vi "HFRR ADV v039 new software.vi"() -> ()   [LabVIEW 2025] (continued)
    n1685 = Fract/Exp String To Number(string=w2065) -> (number=w2064:dbl[])  [unwired: 3 in, 1 out]
    n1686 = call <vilib>:"Median Filter PtByPt.vi"("rank"=2, "x"=w2050) -> ("Filtered x"=→"Friction":dbl)  [unwired: 2 in, 1 out]
    n1687 = Index Array(array=w2064) -> (element #1=→"Sample Temperature":dbl, element #2=→"Target Sample Temperature":dbl, element #3=→"Current Duty Cycle":dbl, element #4=→"Ambient Temperature":dbl, element #5=→"Dac Status":dbl, element #6=→"Vpp":dbl, element #7=→"Active Error Code":dbl, element #8=→"Kp":dbl, element #9=→"Ki":dbl, element #10=→"Kd":dbl, element #11=→"SampleRaw":dbl, element #12=→"AmbRaw":dbl)  [unwired: 12 in]
    n1688 = local read "Quit"() -> (w2070:bool)
  }
  n1689 = while {
    shift-right: [w2084] -> w41
    shift-left: _ -> [w2076]
    shift-right: [w2071] -> w40
    shift-left: errorcluster {"status"=FALSE, "code"=0, "source"="Init"} ("error out") -> [w2078]
    tunnel: [w2073] -> w44
    tunnel: [w2083] -> _
    i -> [w2083]
    stop <- w2073 stop-if-true
    n1690 = local read "Com Port 2"() -> (w2077:refnum<visa-resource-name>)
    n1691 = local read "Port 2a"() -> (w2079:bool)
    n1692 = Unbundle(w2078) -> ("status"=→"Port 4":bool)  [unwired: 2 out]
    n1693 = call <vilib>:"High Resolution Polling Wait.vi"("seconds to wait"=0.02) -> ()  [unwired: 10 in, 1 out]
    n1694 = local read "Port 4"() -> (w2080:bool)
    n1695 = Not Equal?(x=w2077, y=w2076) -> (x != y?=w2075:bool)
    n1696 = Or(x=w2080, y=w2079) -> (x .or. y?=w2082:bool)
    n1697 = case shown="False" w2082 {
      frame False {
        w2087 = TRUE ("Visible")
        n1698 = property on="Port 2a" class="Bool (strict)"("Visible"=w2087) -> ()  [unwired: 2 in, 2 out]
        n1699 = property on="Port 4" class="Bool (strict)"("Visible"=w2087) -> ()  [unwired: 2 in, 2 out]
      }
      frame True {
        w2088 = TRUE ("Visible")
        n1700 = property on="Port 2a" class="Bool (strict)"("Visible"=w2088) -> ()  [unwired: 2 in, 2 out]
        n1701 = property on="Port 4" class="Bool (strict)"("Visible"=w2088) -> ()  [unwired: 2 in, 2 out]
      }
    }
    n1702 = case shown="True" w2075 {
      tunnel: [w2085 errorcluster {"status"=TRUE, "code"=0, "source"="Init"} ("error out")] -> w2074
      tunnel: w2078 -> [w2085 _]
      frame False {
      }
      frame True {
      }
    }
    n1703 = case shown="No Error" w2074 {
      selector: w2074 -> [w2101 w2132]
      tunnel: [w2094 w2137] -> w2084
      tunnel: [w2102 w2130] -> w2071
      tunnel: w2076 -> [w2103 w2135]
      frame No Error {
        n1704 = property class="Instr" props=["Serial Settings:Number of Bytes at Serial Port"](reference=w2103, error in=w2101) -> (reference out=w2095:refnum<visa-resource-name>, error out=w2100:errorcluster)  [unwired: 1 out]
        n1705 = while {
          tunnel: [w2111] -> w2096
          tunnel: [w2110] -> w2097
          tunnel: w2100 -> [w2109]
          tunnel: w2095 -> [w2108]
          tunnel: [w2107] -> _
          i -> [w2107]
          stop <- TRUE stop-if-true
          n1706 = property class="Instr" props=["Serial Settings:Number of Bytes at Serial Port"](reference=w2108, error in=w2109) -> (reference out=w2113:refnum<visa-resource-name>, error out=w2112:errorcluster)  [unwired: 1 out]
          n1707 = VISA Read(VISA resource name=w2113, byte count=u32 1000, error in (no error)=w2112) -> (VISA resource name out=w2110:refnum<visa-resource-name>, read buffer=→"Due read":string, error out=w2111:errorcluster)  [unwired: 1 out]
        }
        n1708 = local read "Due Write"() -> (w2093:string)
        n1709 = call <vilib>:"Trim Whitespace.vi"("string"=w2093) -> ("trimmed string"=w2092:string)  [unwired: 1 in]
        n1710 = Not Equal?(x=w2092, y="") -> (x != y?=w2098:bool)
        n1711 = VISA Flush I/O Buffer(VISA resource name=w2097) -> (VISA resource name out=w2090:refnum<visa-resource-name>, error out=→"error out 10":errorcluster)  [unwired: 2 in]
        n1712 = case shown="True" w2098 {
          tunnel: w2090 -> [w2115 w2120]
          tunnel: [w2115 w2124] -> w2094
          tunnel: w2096 -> [w2114 w2119]
          tunnel: [w2114 w2122] -> w2102
          tunnel: w2092 -> [_ w2118]
          tunnel: [_ w2121] -> _
          frame False {
            # "DATA  WRITE LOOP"
          }
          frame True {
            n1713 = Concatenate Strings(w2118, "\r\n") -> (w2117:string)
            n1714 = VISA Write(VISA resource name=w2120, write buffer=w2117, error in (no error)=w2119) -> (VISA resource name out=w2124:refnum<visa-resource-name>, return count=w2121:u32, error out=w2123:errorcluster)
            n1715 = flat-sequence {
              tunnel: w2123 -> [w2126]
              tunnel: [w2126] -> w2122
              frame #0 {
                n1716 = local write "Due Write"("" ("Command")) -> ()
                n1717 = Wait (ms)(milliseconds to wait=u32 5) -> ()  [unwired: 1 out]
              }
            }
          }
        }
        "Port 2a" <- TRUE ("Port 2a")
      }
      frame Error {
        w2143 = u16 0 items=["None", "XON/XOFF", "RTS/CTS", "XON/XOFF & RTS/CTS", "DTR/DSR", "XON/XOFF & DTR/DSR"] ("flow control (0:none)  2")
        w2141 = u16 10 items=["1.0"=10, "1.5"=15, "2.0"=20] ("stop bits 2")
        w2139 = u16 0 items=["None", "Odd", "Even", "Mark", "Space"] ("parity 2")
        w2140 = u32 10000  # timeout (10sec)
        n1718 = VISA Clear(VISA resource name=w2135, error in (no error)=w2132) -> (VISA resource name out=w2134:refnum<visa-resource-name>, error out=w2133:errorcluster)
        n1719 = VISA Close(VISA resource name=w2134, error in (no error)=w2133) -> (error out=w2136:errorcluster)
        n1720 = call <vilib>:"Clear Errors.vi"("error in (no error)"=w2136) -> ()  [unwired: 5 in, 2 out]
        n1721 = local write "Port 2a"(FALSE ("Port 2a")) -> ()
        n1722 = local read "Com Port 2"() -> (w2129:refnum<visa-resource-name>)
        "visa due" <- w2129
        n1723 = call-poly "VISA Configure Serial Port"("VISA resource name"=w2129, "timeout (10sec)"=w2140, "baud rate (9600)"=u32 250000 ("baud rate  2"), "data bits (8)"=u16 8 ("data bits  2"), "parity (0:none)"=w2139, "stop bits (10: 1 bit)"=w2141, "flow control (0:none)"=w2143) -> ("VISA resource name out"=w2144:refnum<visa-resource-name>, "error out"=w2145:errorcluster)  [unwired: 7 in]
        n1724 = flat-sequence {
          tunnel: w2144 -> [w2147]
          tunnel: w2145 -> [w2146]
          tunnel: [w2147] -> w2137
          tunnel: [w2146] -> w2130
          frame #0 {
            n1725 = Wait (ms)(milliseconds to wait=u32 50) -> ()  [unwired: 1 out]
          }
        }
        "Residual Due" <- ""
      }
    }
    "error out 9" <- w2071
    n1726 = local read "Quit"() -> (w2073:bool)
    "Error Due" <- w2078
  }
  n1727 = local write "FRICVALZ"(0.0 ("FRICVALZ")) -> ()
  n1728 = property on="RUN" class="Bool (strict)"("Visible"=TRUE) -> ()  [unwired: 2 in, 2 out]
  n1729 = while {
    tunnel: [w2162] -> _
    tunnel: [w2149] -> w54
    i -> [w2162]
    stop <- w2149 stop-if-true
    # "DATA PROCESSING"
    # "115 mV/N"
    n1730 = local read "conststatus"() -> (w2153:dbl)
    n1731 = local read "Main Tab"() -> (w2151:T2)
    n1732 = local read "EDIT"() -> (w2168:bool)
    n1733 = local read "Rate"() -> (w2167:dbl)
    n1734 = case shown="True" w2168 {
      tunnel: [FALSE TRUE] -> _
      frame False {
      }
      frame True {
      }
    }
    n1735 = Equal?(x=w2151, y=T29."About" ("Main Tab")) -> (x = y?=w2160:bool)
    n1736 = Equal?(x=w2153, y=0.0) -> (x = y?=w2154:bool)
    n1737 = Divide(x=1.0, y=w2167) -> (x/y=w2163:dbl)
    "Time 2" <- w2163
    n1738 = case shown="True" w2154 {
      frame False {
      }
      frame True {
        # "C:\\WinDucom\\calibrate WO 2391.dcf"
        n1739 = local write "Lan flag"(22) -> ()
        n1740 = local write "conststatus"(10.0 ("rpm value : 2")) -> ()
        n1741 = String To Path(string="C:\\LAB-IQ\\calibrate WO 2465.dcf") -> (path=w2174:path)
        n1742 = Open/Create/Replace File "Open File"(file path (use dialog)=w2174) -> (refnum out=w2172:refnum<file>)  [unwired: 5 in, 2 out]
        n1743 = for {
          N: 23 -> [_]
          tunnel: w2172 -> [w2183]
          i -> [w2177]
          (unwired) TRUE ("line mode (F)")
          n1744 = Read from Text File "Read File"(file (use dialog)=w2183) -> (text=w2182:string)  [unwired: 3 in, 3 out]
          n1745 = Match Pattern(string=w2182, regular expression="]") -> (after substring=w2180:string)  [unwired: 1 in, 3 out]
          n1746 = String Subset(string=w2182, offset (0)=5, length (rest)=10 ("length (rest)")) -> (substring=w2175:string)
          n1747 = Fract/Exp String To Number(string=w2175) -> (number=w2176:dbl)  [unwired: 3 in, 1 out]
          n1748 = Match Pattern(string=w2180, regular expression="-") -> (before substring=w2178:string)  [unwired: 1 in, 3 out]
          n1749 = case shown="10" w2177 {
            tunnel: w2176 -> [_ _ _ _ _ _ _ _ _ _ w2190 _ _ _ _ _ _ _ _ _ _ _ _ _]
            tunnel: w2178 -> [_ _ _ _ w2186 w2187 w2188 _ _ _ _ _ _ _ _ _ _ _ _ _ w2191 w2192 w2193 _]
            frame 0 {
            }
            frame 1 {
            }
            frame 2 {
            }
            frame 3 {
            }
            frame 4 {
              n1750 = local write "Com Port 1"(w2186) -> ()
            }
            frame 5 {
              n1751 = local write "Com Port 2"(w2187) -> ()
              n1752 = local write "visa due"(w2187) -> ()
            }
            frame 6 {
              n1753 = String To Path(string=w2188) -> (path=w2189:path)
              n1754 = local write "File Path"(w2189) -> ()
              "String" <- w2188
            }
            frame 7 {
            }
            frame 8 {
            }
            frame 9 {
            }
            frame 10 {
              n1755 = local write "Language Selection"(w2190) -> ()
            }
            frame 11 {
            }
            frame 12 {
            }
            frame 13 {
            }
            frame 14 {
            }
            frame 15 {
            }
            frame 16 {
            }
            frame 17 {
            }
            frame 18 {
            }
            frame 21 {
            }
            frame 22 {
              n1756 = local write "Com Port 3"(w2191) -> ()
            }
            frame 20 {
              n1757 = local write "Camera Port :"(w2192) -> ()
            }
            frame 19 {
              n1758 = local write "C3 :"(w2193) -> ()
            }
            frame 23, Default {
            }
          }
        }
      }
    }
    n1759 = Select(t=u32 2500 ("milliseconds to wait"), s=w2160, f=u32 500 ("milliseconds to wait")) -> (s? t:f=w2158:u32)
    n1760 = Multiply(x=w2163, y=w2158) -> (x*y=w2165:dbl)
    n1761 = call "Elapsed Time2"("Time Target (s)"=w2165, "Auto Reset"=TRUE) -> ("Time has Elapsed"=w2155:bool)  [unwired: 10 in, 7 out]
    n1762 = case shown="True" w2155 {
      frame False {
      }
      frame True {
        n1763 = stacked-sequence {
          frame #0 {
            n1764 = local read "Sample Temperature"() -> (w2197:dbl)
            n1765 = local read "RH Numeric:"() -> (→"Humidity ( %RH )" →"Hum":dbl)
            n1766 = local read "FF CONTINUE 5"() -> (w2194:bool)
            n1767 = local read "FRICVALZ"() -> (w2214:dbl)
            n1768 = local read "Friction"() -> (w2200:dbl)
            n1769 = call <vilib>:"Mean PtByPt.vi"("x"=w2197, "sample length"=100) -> ("mean"=w2196:dbl)  [unwired: 2 in, 1 out]
            "TEMP 2" <- w2196
            "TEMP 3" <- w2196
            n1770 = Subtract(x=w2200, y=w2214) -> (x-y=w2209:dbl)
            "FF 2" <- w2209
            "FF 4" <- w2209
            n1771 = local read "Ambient Temperature"() -> (→"AIR TEMP":dbl)
            n1772 = local read "TEMP"() -> (w2213:dbl)
            n1773 = local write "FF 3"(w2209) -> ()
            n1774 = Compound Arithmetic op=OR("FRICVALZ 4", "FRICVALZ 3", "FRICVALZ 2", w2194) -> (w2205:bool)
            n1775 = case shown="True" w2205 {
              tunnel: w2200 -> [_ w2220]
              frame False {
              }
              frame True {
                w2219 = FALSE ("FRICVALZ")
                n1776 = local write "FRICVALZ 3"(w2219) -> ()
                n1777 = local write "FRICVALZ 2"(w2219) -> ()
                n1778 = local write "FRICVALZ 4"(w2219) -> ()
                n1779 = local write "FF CONTINUE 5"(w2219) -> ()
                "FRICVALZ" <- w2220
              }
            }
            n1780 = Not A Number/Path/Refnum?(number/path/refnum=w2213) -> (NaN/Path/Refnum?=w2212:bool)
            n1781 = Not A Number/Path/Refnum?(number/path/refnum=w2209) -> (NaN/Path/Refnum?=w2211:bool)
            n1782 = Divide(x=w2209, y=1.96) -> (x/y=w2206:dbl)
            n1783 = Compound Arithmetic op=OR(w2212, w2211) -> (w2210:bool)
            n1784 = Not A Number/Path/Refnum?(number/path/refnum=w2206) -> (NaN/Path/Refnum?=w2207:bool)
            n1785 = case shown="True" w2210 {
              frame False {
              }
              frame True {
                n1786 = local write "TEMP"(0.0 ("TEMP")) -> ()
                n1787 = local write "FF 2"(0.0 ("FF 2")) -> ()
                n1788 = local write "reinit"(TRUE ("reinit")) -> ()
              }
            }
            n1789 = local write "TEMP"(w2196) -> ()
            n1790 = Select(t=0.0, s=w2207, f=w2206) -> (s? t:f=w2199:dbl)
            "COF 2" <- w2199
            n1791 = local write "COF 3"(w2199) -> ()
          }
        }
      }
    }
    n1792 = Wait (ms)(milliseconds to wait=u32 50) -> ()  [unwired: 1 out]
    n1793 = local read "Quit"() -> (w2149:bool)
    "Rate" <- 2500.0 ("No of Samples")
  }
  n1794 = VISA Close(VISA resource name=w41, error in (no error)=w40) -> ()  [unwired: 1 out]
  n1795 = while {
    tunnel: [w2240] -> _
    tunnel: [w2223] -> w56
    tunnel: w1 -> [_]
    i -> [w2240]
    stop <- w2223 stop-if-true
    # "C:\\LAB-IQ-NXT\\Scar View.exe"
    n1796 = local read "OK Button 16"() -> (w2230:bool)
    n1797 = local read "Main Tab"() -> (w2224:T2)
    n1798 = local read "service 3"() -> (w2225:bool)
    n1799 = local read "OPEN 6"() -> (w2227:bool)
    n1800 = local read "EDIT 2"() -> (w2229:bool)
    n1801 = local read "RUN"() -> (w2237:bool)
    n1802 = local read "RUN"() -> (w2239:bool)
    n1803 = case shown="True" "EDIT 3" {
      frame False {
      }
      frame True {
        n1804 = local write "EDIT 3"(FALSE ("EDIT 3")) -> ()
        n1805 = local write "Main Tab"(T2."About" ("Main Tab")) -> ()
      }
    }
    n1806 = case shown="\"ISO 12156\"" "TEST STANDARD" {
      frame "ASTM D6079", Default {
        w2674 = 50.0 ("Hz")
        w2675 = 53.0 ("Set Rh")
        w2677 = 1.0 ("Set Strk")
        w2676 = 60.0 ("Set Temp")
        # "astm hide"
        n1807 = local write "NORMAL LOAD"(200.0 ("NORMAL LOAD")) -> ()
        n1808 = local write "Set Strk"(w2677) -> ()
        n1809 = local write "Set Hz"(w2674) -> ()
        n1810 = local write "test time"(75.0 ("test time")) -> ()
        n1811 = local write "Set Rh"(w2675) -> ()
        n1812 = local write "Set Temp"(w2676) -> ()
        n1813 = local write "Set Stroke:"(w2677) -> ()
        n1814 = local write "Set Humidity:"(w2675) -> ()
        n1815 = local write "Set Frequency:"(w2674) -> ()
        n1816 = local write "Set Temperature:"(w2676) -> ()
        "Test Standard" <- "ASTM D6079" ("Test Standard 2")
      }
      frame "ISO 12156" {
        n1817 = local write "NORMAL LOAD"(200.0 ("NORMAL LOAD")) -> ()
        n1818 = local write "Set Strk"(1.0 ("Set Strk")) -> ()
        n1819 = local write "Set Hz"(50.0 ("Hz")) -> ()
        n1820 = local write "test time"(75.0 ("test time")) -> ()
        n1821 = local write "Set Rh"(53.0 ("Set Rh")) -> ()
        n1822 = local write "Set Temp"(60.0 ("Set Temp")) -> ()
      }
      frame "CEC F-096-A-06" {
        n1823 = local write "NORMAL LOAD"(200.0 ("NORMAL LOAD")) -> ()
        n1824 = local write "Set Strk"(1.0 ("Set Strk")) -> ()
        n1825 = local write "Set Hz"(50.0 ("Hz")) -> ()
        n1826 = local write "test time"(75.0 ("test time")) -> ()
        n1827 = local write "Set Rh"(53.0 ("Set Rh")) -> ()
        n1828 = local write "Set Temp"(60.0 ("Set Temp")) -> ()
      }
      frame "Custom" {
      }
    }
    n1829 = case shown="False" w2237 {
      frame False {
      }
      frame True {
      }
    }
    n1830 = Or(x=w2227, y=w2225) -> (x .or. y?=w2226:bool)
    n1831 = case shown="\"About\"" w2224 {
      tunnel: [T29."Acquire" ("Main Tab") T29."Compare Files" ("Main Tab") T29."About" ("Main Tab")] -> w2235
      frame "Acquire", Default {
      }
      frame "Compare Files" {
      }
      frame "About" {
      }
    }
    n1832 = Or(x=w2230, y="OPEN") -> (x .or. y?=w2231:bool)
    n1833 = case shown="True" w2231 {
      tunnel: w2230 -> [_ w2263]
      frame False {
      }
      frame True {
        n1834 = stacked-sequence {
          tunnel: w2263 -> [_ w2330 _ _]
          frame #0 {
            w2279 = "  " ("String 6")
            n1835 = local write "OPEN"(FALSE ("open")) -> ()
            n1836 = local read "string1 4"() -> (w2265:string)
            n1837 = local read "string1 3"() -> (w2266:string)
            n1838 = local read "string1 2"() -> (w2267:string)
            n1839 = local write "String 6"(w2279) -> ()
            n1840 = local write "String 7"(w2279) -> ()
            n1841 = local write "String 8"(w2279) -> ()
            n1842 = local write "String 12"(w2279) -> ()
            n1843 = property on="OPEN" class="Bool (strict)"("Visible"=FALSE) -> ()  [unwired: 2 in, 2 out]
            n1844 = local read "OK Button 16"() -> (w2264:bool)
            n1845 = String To Path(string=w2265) -> (path=w2273:path)
            n1846 = String To Path(string=w2266) -> (path=w2274:path)
            n1847 = String To Path(string=w2267) -> (path=w2275:path)
            n1848 = case shown="True" w2264 {
              tunnel: [w2280 w2281] -> w2268
              frame False {
                n1849 = local read "string1"() -> (w2280:string)
              }
              frame True {
                n1850 = local read "String Indicator 4"() -> (w2281:string)
              }
            }
            n1851 = Open/Create/Replace File "Open File"(file path (use dialog)=w2275) -> (refnum out=w2271:refnum<file>)  [unwired: 5 in, 2 out]
            n1852 = Open/Create/Replace File "Open File"(file path (use dialog)=w2274) -> (refnum out=w2270:refnum<file>)  [unwired: 5 in, 2 out]
            n1853 = Open/Create/Replace File "Open File"(file path (use dialog)=w2273) -> (refnum out=w2269:refnum<file>)  [unwired: 5 in, 2 out]
            n1854 = while {
              tunnel: w2271 -> [w2293]
              i -> [w2289]
              stop <- w2288 continue-if-true
              (unwired) TRUE ("line mode (F)")
              n1855 = Read from Text File "Read File"(file (use dialog)=w2293) -> (text=w2290:string)  [unwired: 3 in, 3 out]
              n1856 = local write "Numeric 11"(w2289) -> ()
              n1857 = String Length(string=w2290) -> (length=w2292:i32)
              n1858 = Greater?(x=w2292, y=1) -> (0:w2288:bool)
            }
            n1859 = while {
              tunnel: w2270 -> [w2299]
              i -> [w2295]
              stop <- w2294 continue-if-true
              (unwired) TRUE ("line mode (F)")
              n1860 = Read from Text File "Read File"(file (use dialog)=w2299) -> (text=w2296:string)  [unwired: 3 in, 3 out]
              n1861 = local write "Numeric 12"(w2295) -> ()
              n1862 = String Length(string=w2296) -> (length=w2298:i32)
              n1863 = Greater?(x=w2298, y=1) -> (0:w2294:bool)
            }
            n1864 = while {
              tunnel: w2269 -> [w2305]
              i -> [w2301]
              stop <- w2300 continue-if-true
              (unwired) TRUE ("line mode (F)")
              n1865 = Read from Text File "Read File"(file (use dialog)=w2305) -> (text=w2302:string)  [unwired: 3 in, 3 out]
              n1866 = local write "Numeric 13"(w2301) -> ()
              n1867 = String Length(string=w2302) -> (length=w2304:i32)
              n1868 = Greater?(x=w2304, y=1) -> (0:w2300:bool)
            }
            n1869 = String To Path(string=w2268) -> (path=w2276:path)
            n1870 = Open/Create/Replace File "Open File"(file path (use dialog)=w2276) -> (refnum out=w2272:refnum<file>)  [unwired: 5 in, 2 out]
            n1871 = while {
              tunnel: w2272 -> [w2287]
              i -> [w2283]
              stop <- w2282 continue-if-true
              (unwired) TRUE ("line mode (F)")
              n1872 = Read from Text File "Read File"(file (use dialog)=w2287) -> (text=w2284:string)  [unwired: 3 in, 3 out]
              n1873 = local write "Numeric 8"(w2283) -> ()
              n1874 = String Length(string=w2284) -> (length=w2286:i32)
              n1875 = Greater?(x=w2286, y=1) -> (0:w2282:bool)
            }
          }
          frame #1 {
            w2457 = FALSE ("ACTUAL   MERGE")
            # "Sample Temp"
            # "ECR"
            # "COF"
            # "Time\nCOF\nFF\nTemp"
            n1876 = case shown="True" w2330 {
              tunnel: [w2477 w2478] -> w2331
              frame False {
                n1877 = local read "string1"() -> (w2477:string)
              }
              frame True {
                n1878 = local read "String Indicator 4"() -> (w2478:string)
              }
            }
            n1879 = local read "string1 3"() -> (w2375:string)
            n1880 = String To Path(string=w2375) -> (path=w2473:path)
            n1881 = String To Path(string=w2331) -> (path=w2462:path)
            n1882 = local read "Numeric 12"() -> (w2459:i32)
            n1883 = local read "Numeric 8"() -> (w2461:i32)
            n1884 = local read "string1 4"() -> (w2374:string)
            n1885 = local read "string1 2"() -> (w2376:string)
            n1886 = Open/Create/Replace File "Open File"(file path (use dialog)=w2462) -> (refnum out=w2476:refnum<file>, error out=w2475:errorcluster)  [unwired: 5 in, 1 out]
            n1887 = Open/Create/Replace File "Open File"(file path (use dialog)=w2473) -> (refnum out=w2469:refnum<file>, error out=w2470:errorcluster)  [unwired: 5 in, 1 out]
            n1888 = for {
              N: w2459 -> [_]
              tunnel: w2470 -> [w2550]
              tunnel: w2469 -> [w2549]
              tunnel: [w2539] -> w2428 mode=indexing
              tunnel: [w2537] -> w2426 mode=indexing
              tunnel: [w2538] -> w2422 mode=indexing
              tunnel: w2457 -> [_]
              tunnel: [w2531] -> w2424 mode=indexing
              tunnel: [w2527] -> w2406 mode=indexing
              tunnel: [w2523] -> w2382 mode=indexing
              tunnel: [w2520] -> w2363 mode=indexing
              tunnel: [w2516] -> w2322 mode=indexing
              (unwired) 9 ("length (rest)")
              (unwired) 9 ("length (rest)")
              (unwired) TRUE ("line mode (F)")
              n1889 = Read from Text File "Read File"(file (use dialog)=w2549, error in=w2550) -> (text=w2517:string)  [unwired: 2 in, 3 out]
              n1890 = local write "String 8"(w2517) -> ()
              n1891 = String Subset(string=w2517, offset (0)=85) -> (substring=w2519:string)  [unwired: 1 in]
              n1892 = String Subset(string=w2517, offset (0)=25) -> (substring=w2521:string)  [unwired: 1 in]
              n1893 = String Subset(string=w2517, offset (0)=55, length (rest)=9 ("length (rest)")) -> (substring=w2525:string)
              n1894 = String Subset(string=w2517, offset (0)=45, length (rest)=9 ("length (rest)")) -> (substring=w2530:string)
              n1895 = String Subset(string=w2517, offset (0)=65, length (rest)=9 ("length (rest)")) -> (substring=w2536:string)
              n1896 = String Subset(string=w2517, offset (0)=35, length (rest)=9 ("length (rest)")) -> (substring=w2540:string)
              n1897 = String Subset(string=w2517, offset (0)=0, length (rest)=14 ("length (rest)")) -> (substring=w2543:string)
              n1898 = String Subset(string=w2517, offset (0)=15, length (rest)=9 ("length (rest)")) -> (substring=w2546:string)
              n1899 = Fract/Exp String To Number(string=w2519) -> (number=w2516:dbl)  [unwired: 3 in, 1 out]
              n1900 = Fract/Exp String To Number(string=w2521) -> (number=w2520:dbl)  [unwired: 3 in, 1 out]
              n1901 = Fract/Exp String To Number(string=w2525) -> (number=w2523:dbl)  [unwired: 3 in, 1 out]
              n1902 = Fract/Exp String To Number(string=w2530) -> (number=w2527:dbl)  [unwired: 3 in, 1 out]
              n1903 = Fract/Exp String To Number(string=w2536) -> (number=w2533:dbl)  [unwired: 3 in, 1 out]
              n1904 = Fract/Exp String To Number(string=w2540) -> (number=w2538:dbl)  [unwired: 3 in, 1 out]
              n1905 = Fract/Exp String To Number(string=w2543) -> (number=w2539:dbl)  [unwired: 3 in, 1 out]
              n1906 = Fract/Exp String To Number(string=w2546) -> (number=w2537:dbl)  [unwired: 3 in, 1 out]
              n1907 = Add(x=w2533, y=0.0) -> (x+y=w2531:dbl)
            }
            n1908 = for {
              N: w2461 -> [_]
              tunnel: w2476 -> [w2624]
              tunnel: w2475 -> [w2623]
              tunnel: [w2613] -> w2388 mode=indexing
              tunnel: [w2611] -> w2445 mode=indexing
              tunnel: [w2612] -> w2440 mode=indexing
              tunnel: w2457 -> [_]
              tunnel: [w2605] -> w2442 mode=indexing
              tunnel: [w2601] -> w2411 mode=indexing
              tunnel: [w2597] -> w2386 mode=indexing
              tunnel: [w2593] -> w2367 mode=indexing
              tunnel: [w2588] -> w2327 mode=indexing
              (unwired) TRUE ("line mode (F)")
              # "freq"
              # "Stroke"
              # "Time"
              # "CoF"
              # "Humidity"
              # "Temp"
              # "Air Temp"
              # "ECR"
              n1909 = Read from Text File "Read File"(file (use dialog)=w2624, error in=w2623) -> (text=w2589:string)  [unwired: 2 in, 3 out]
              n1910 = local write "String 6"(w2589) -> ()
              n1911 = String Subset(string=w2589, offset (0)=35, length (rest)=9 ("length (rest)")) -> (substring=w2614:string)
              n1912 = String Subset(string=w2589, offset (0)=0, length (rest)=14 ("length (rest)")) -> (substring=w2617:string)
              n1913 = String Subset(string=w2589, offset (0)=15, length (rest)=9 ("length (rest)")) -> (substring=w2620:string)
              n1914 = Fract/Exp String To Number(string=w2614) -> (number=w2612:dbl)  [unwired: 3 in, 1 out]
              n1915 = Fract/Exp String To Number(string=w2617) -> (number=w2613:dbl)  [unwired: 3 in, 1 out]
              n1916 = Fract/Exp String To Number(string=w2620) -> (number=w2611:dbl)  [unwired: 3 in, 1 out]
              n1917 = String Subset(string=w2589, offset (0)=85, length (rest)=9 ("length (rest)")) -> (substring=w2590:string)
              n1918 = String Subset(string=w2589, offset (0)=25, length (rest)=9 ("length (rest)")) -> (substring=w2596:string)
              n1919 = String Subset(string=w2589, offset (0)=55, length (rest)=9 ("length (rest)")) -> (substring=w2598:string)
              n1920 = String Subset(string=w2589, offset (0)=45, length (rest)=9 ("length (rest)")) -> (substring=w2604:string)
              n1921 = String Subset(string=w2589, offset (0)=65, length (rest)=9 ("length (rest)")) -> (substring=w2610:string)
              n1922 = Fract/Exp String To Number(string=w2596) -> (number=w2593:dbl)  [unwired: 3 in, 1 out]
              n1923 = Fract/Exp String To Number(string=w2590) -> (number=w2588:dbl)  [unwired: 3 in, 1 out]
              n1924 = Fract/Exp String To Number(string=w2598) -> (number=w2597:dbl)  [unwired: 3 in, 1 out]
              n1925 = Fract/Exp String To Number(string=w2604) -> (number=w2601:dbl)  [unwired: 3 in, 1 out]
              n1926 = Fract/Exp String To Number(string=w2610) -> (number=w2607:dbl)  [unwired: 3 in, 1 out]
              n1927 = Add(x=w2607, y=0.0) -> (x+y=w2605:dbl)
            }
            n1928 = String To Path(string=w2374) -> (path=w2468:path)
            n1929 = String To Path(string=w2376) -> (path=w2474:path)
            n1930 = local read "Numeric 11"() -> (w2458:i32)
            n1931 = local read "Numeric 13"() -> (w2460:i32)
            n1932 = Open/Create/Replace File "Open File"(file path (use dialog)=w2474) -> (refnum out=w2472:refnum<file>, error out=w2471:errorcluster)  [unwired: 5 in, 1 out]
            n1933 = Open/Create/Replace File "Open File"(file path (use dialog)=w2468) -> (refnum out=w2467:refnum<file>, error out=w2466:errorcluster)  [unwired: 5 in, 1 out]
            n1934 = for {
              N: w2460 -> [_]
              tunnel: w2467 -> [w2515]
              tunnel: w2466 -> [w2514]
              tunnel: [w2504] -> w2420 mode=indexing
              tunnel: [w2503] -> w2413 mode=indexing
              tunnel: w2457 -> [_]
              tunnel: [w2492] -> w2418 mode=indexing
              tunnel: [w2497] -> w2415 mode=indexing
              tunnel: [w2493] -> w2405 mode=indexing
              tunnel: [w2488] -> w2380 mode=indexing
              tunnel: [w2484] -> w2361 mode=indexing
              tunnel: [w2479] -> w2321 mode=indexing
              (unwired) 1.0 ("x")
              (unwired) TRUE ("line mode (F)")
              n1935 = Read from Text File "Read File"(file (use dialog)=w2515, error in=w2514) -> (text=w2480:string)  [unwired: 2 in, 3 out]
              n1936 = local write "String 12"(w2480) -> ()
              n1937 = String Subset(string=w2480, offset (0)=85, length (rest)=9 ("length (rest)")) -> (substring=w2482:string)
              n1938 = String Subset(string=w2480, offset (0)=25, length (rest)=9 ("length (rest)")) -> (substring=w2486:string)
              n1939 = String Subset(string=w2480, offset (0)=55, length (rest)=9 ("length (rest)")) -> (substring=w2490:string)
              n1940 = String Subset(string=w2480, offset (0)=45, length (rest)=9 ("length (rest)")) -> (substring=w2495:string)
              n1941 = String Subset(string=w2480, offset (0)=65, length (rest)=9 ("length (rest)")) -> (substring=w2498:string)
              n1942 = String Subset(string=w2480, offset (0)=35, length (rest)=9 ("length (rest)")) -> (substring=w2505:string)
              n1943 = String Subset(string=w2480, offset (0)=0, length (rest)=14 ("length (rest)")) -> (substring=w2508:string)
              n1944 = String Subset(string=w2480, offset (0)=15, length (rest)=9 ("length (rest)")) -> (substring=w2511:string)
              n1945 = Fract/Exp String To Number(string=w2482) -> (number=w2479:dbl)  [unwired: 3 in, 1 out]
              n1946 = Fract/Exp String To Number(string=w2486) -> (number=w2484:dbl)  [unwired: 3 in, 1 out]
              n1947 = Fract/Exp String To Number(string=w2490) -> (number=w2488:dbl)  [unwired: 3 in, 1 out]
              n1948 = Fract/Exp String To Number(string=w2495) -> (number=w2493:dbl)  [unwired: 3 in, 1 out]
              n1949 = Fract/Exp String To Number(string=w2498) -> (number=w2501:dbl)  [unwired: 3 in, 1 out]
              n1950 = Fract/Exp String To Number(string=w2505) -> (number=w2503:dbl)  [unwired: 3 in, 1 out]
              n1951 = Fract/Exp String To Number(string=w2508) -> (number=w2504:dbl)  [unwired: 3 in, 1 out]
              n1952 = Fract/Exp String To Number(string=w2511) -> (number=w2492:dbl)  [unwired: 3 in, 1 out]
              n1953 = Add(x=w2501, y=0.0) -> (x+y=w2497:dbl)
            }
            n1954 = for {
              N: w2458 -> [_]
              tunnel: w2472 -> [w2587]
              tunnel: w2471 -> [w2586]
              tunnel: [w2576] -> w2438 mode=indexing
              tunnel: [w2574] -> w2436 mode=indexing
              tunnel: [w2575] -> w2431 mode=indexing
              tunnel: w2457 -> [_]
              tunnel: [w2568] -> w2433 mode=indexing
              tunnel: [w2564] -> w2409 mode=indexing
              tunnel: [w2560] -> w2384 mode=indexing
              tunnel: [w2556] -> w2365 mode=indexing
              tunnel: [w2551] -> w2323 mode=indexing
              (unwired) TRUE ("line mode (F)")
              n1955 = Read from Text File "Read File"(file (use dialog)=w2587, error in=w2586) -> (text=w2552:string)  [unwired: 2 in, 3 out]
              n1956 = local write "String 7"(w2552) -> ()
              n1957 = String Subset(string=w2552, offset (0)=85, length (rest)=9 ("length (rest)")) -> (substring=w2555:string)
              n1958 = String Subset(string=w2552, offset (0)=25, length (rest)=9 ("length (rest)")) -> (substring=w2557:string)
              n1959 = String Subset(string=w2552, offset (0)=55, length (rest)=9 ("length (rest)")) -> (substring=w2563:string)
              n1960 = String Subset(string=w2552, offset (0)=45, length (rest)=9 ("length (rest)")) -> (substring=w2565:string)
              n1961 = String Subset(string=w2552, offset (0)=65, length (rest)=9 ("length (rest)")) -> (substring=w2569:string)
              n1962 = String Subset(string=w2552, offset (0)=35, length (rest)=9 ("length (rest)")) -> (substring=w2577:string)
              n1963 = String Subset(string=w2552, offset (0)=0, length (rest)=14 ("length (rest)")) -> (substring=w2580:string)
              n1964 = String Subset(string=w2552, offset (0)=15, length (rest)=9 ("length (rest)")) -> (substring=w2583:string)
              n1965 = Fract/Exp String To Number(string=w2555) -> (number=w2551:dbl)  [unwired: 3 in, 1 out]
              n1966 = Fract/Exp String To Number(string=w2557) -> (number=w2556:dbl)  [unwired: 3 in, 1 out]
              n1967 = Fract/Exp String To Number(string=w2563) -> (number=w2560:dbl)  [unwired: 3 in, 1 out]
              n1968 = Fract/Exp String To Number(string=w2565) -> (number=w2564:dbl)  [unwired: 3 in, 1 out]
              n1969 = Fract/Exp String To Number(string=w2569) -> (number=w2572:dbl)  [unwired: 3 in, 1 out]
              n1970 = Fract/Exp String To Number(string=w2577) -> (number=w2575:dbl)  [unwired: 3 in, 1 out]
              n1971 = Fract/Exp String To Number(string=w2580) -> (number=w2576:dbl)  [unwired: 3 in, 1 out]
              n1972 = Fract/Exp String To Number(string=w2583) -> (number=w2574:dbl)  [unwired: 3 in, 1 out]
              n1973 = Add(x=w2572, y=0.0) -> (x+y=w2568:dbl)
            }
            n1974 = Delete From Array(array=w2363, index=0) -> (array with subset deleted=w2336:dbl[])  [unwired: 1 in, 1 out]
            n1975 = Delete From Array(array=w2406, index=0) -> (array with subset deleted=w2394:dbl[])  [unwired: 1 in, 1 out]
            n1976 = Delete From Array(array=w2424, index=0) -> (array with subset deleted=w2425:dbl[])  [unwired: 1 in, 1 out]
            n1977 = Delete From Array(array=w2426, index=0) -> (array with subset deleted=w2399:dbl[])  [unwired: 1 in, 1 out]
            n1978 = call-poly <vilib>:"Mean.vi"("X"=w2399) -> ("mean"=→"КОФ3":dbl)  [unwired: 1 out]
            n1979 = call-poly <vilib>:"Mean.vi"("X"=w2394) -> ("mean"=→"CP3":dbl)  [unwired: 1 out]
            n1980 = call-poly <vilib>:"Mean.vi"("X"=w2336) -> ("mean"=→"КОФ2 4":dbl)  [unwired: 1 out]
            n1981 = Delete From Array(array=w2327, index=0) -> (array with subset deleted=w2314:dbl[])  [unwired: 1 in, 1 out]
            n1982 = Delete From Array(array=w2367, index=0) -> (array with subset deleted=w2338:dbl[])  [unwired: 1 in, 1 out]
            n1983 = Delete From Array(array=w2411, index=0) -> (array with subset deleted=w2396:dbl[])  [unwired: 1 in, 1 out]
            "array w/ subset deleted" <- w2396
            n1984 = Delete From Array(array=w2442, index=0) -> (array with subset deleted=w2443:dbl[])  [unwired: 1 in, 1 out]
            n1985 = Delete From Array(array=w2445, index=0) -> (array with subset deleted=w2400:dbl[])  [unwired: 1 in, 1 out]
            n1986 = Delete From Array(array=w2388, index=0) -> (array with subset deleted=w2315:dbl[])  [unwired: 1 in, 1 out]
            n1987 = call-poly <vilib>:"Mean.vi"("X"=w2400) -> ("mean"=→"КОФ1":dbl)  [unwired: 1 out]
            n1988 = call-poly <vilib>:"Mean.vi"("X"=w2338) -> ("mean"=→"КОФ2 2":dbl)  [unwired: 1 out]
            n1989 = Bundle "Bundle"(w2315, w2314) -> (w2320:cluster{dbl[], dbl[]})  [unwired: 1 in]
            n1990 = Bundle "Bundle"(w2315, w2443) -> (w2307:cluster{dbl[], dbl[]})  [unwired: 1 in]
            n1991 = Delete From Array(array=w2321, index=0) -> (array with subset deleted=w2308:dbl[])  [unwired: 1 in, 1 out]
            n1992 = Delete From Array(array=w2322, index=0) -> (array with subset deleted=w2310:dbl[])  [unwired: 1 in, 1 out]
            n1993 = Delete From Array(array=w2323, index=0) -> (array with subset deleted=w2312:dbl[])  [unwired: 1 in, 1 out]
            n1994 = Delete From Array(array=w2415, index=0) -> (array with subset deleted=w2416:dbl[])  [unwired: 1 in, 1 out]
            n1995 = Delete From Array(array=w2433, index=0) -> (array with subset deleted=w2434:dbl[])  [unwired: 1 in, 1 out]
            n1996 = Delete From Array(array=w2361, index=0) -> (array with subset deleted=w2335:dbl[])  [unwired: 1 in, 1 out]
            n1997 = Delete From Array(array=w2365, index=0) -> (array with subset deleted=w2337:dbl[])  [unwired: 1 in, 1 out]
            n1998 = Delete From Array(array=w2380, index=0) -> (array with subset deleted=w2339:dbl[])  [unwired: 1 in, 1 out]
            n1999 = Delete From Array(array=w2382, index=0) -> (array with subset deleted=w2340:dbl[])  [unwired: 1 in, 1 out]
            n2000 = Delete From Array(array=w2384, index=0) -> (array with subset deleted=w2341:dbl[])  [unwired: 1 in, 1 out]
            n2001 = Delete From Array(array=w2386, index=0) -> (array with subset deleted=w2342:dbl[])  [unwired: 1 in, 1 out]
            n2002 = Delete From Array(array=w2405, index=0) -> (array with subset deleted=w2393:dbl[])  [unwired: 1 in, 1 out]
            n2003 = Delete From Array(array=w2409, index=0) -> (array with subset deleted=w2395:dbl[])  [unwired: 1 in, 1 out]
            n2004 = Delete From Array(array=w2413, index=0) -> (array with subset deleted=w2343:dbl[])  [unwired: 1 in, 1 out]
            n2005 = Delete From Array(array=w2418, index=0) -> (array with subset deleted=w2398:dbl[])  [unwired: 1 in, 1 out]
            n2006 = Delete From Array(array=w2422, index=0) -> (array with subset deleted=w2344:dbl[])  [unwired: 1 in, 1 out]
            n2007 = Delete From Array(array=w2431, index=0) -> (array with subset deleted=w2345:dbl[])  [unwired: 1 in, 1 out]
            n2008 = Delete From Array(array=w2436, index=0) -> (array with subset deleted=w2397:dbl[])  [unwired: 1 in, 1 out]
            n2009 = Delete From Array(array=w2440, index=0) -> (array with subset deleted=w2346:dbl[])  [unwired: 1 in, 1 out]
            n2010 = Delete From Array(array=w2420, index=0) -> (array with subset deleted=w2309:dbl[])  [unwired: 1 in, 1 out]
            n2011 = Delete From Array(array=w2428, index=0) -> (array with subset deleted=w2311:dbl[])  [unwired: 1 in, 1 out]
            n2012 = Delete From Array(array=w2438, index=0) -> (array with subset deleted=w2313:dbl[])  [unwired: 1 in, 1 out]
            n2013 = Bundle "Bundle"(w2309, w2308) -> (w2317:cluster{dbl[], dbl[]})  [unwired: 1 in]
            n2014 = Bundle "Bundle"(w2311, w2310) -> (w2318:cluster{dbl[], dbl[]})  [unwired: 1 in]
            n2015 = Bundle "Bundle"(w2313, w2312) -> (w2319:cluster{dbl[], dbl[]})  [unwired: 1 in]
            n2016 = Bundle "Bundle"(w2343, w2339) -> (w2351:cluster{dbl[], dbl[]})  [unwired: 1 in]
            n2017 = Bundle "Bundle"(w2344, w2340) -> (w2350:cluster{dbl[], dbl[]})  [unwired: 1 in]
            n2018 = Bundle "Bundle"(w2345, w2341) -> (w2349:cluster{dbl[], dbl[]})  [unwired: 1 in]
            n2019 = Bundle "Bundle"(w2346, w2342) -> (w2348:cluster{dbl[], dbl[]})  [unwired: 1 in]
            n2020 = Bundle "Bundle"(w2309, w2339) -> (w2377:cluster{dbl[], dbl[]})  [unwired: 1 in]
            n2021 = Bundle "Bundle"(w2311, w2340) -> (w2378:cluster{dbl[], dbl[]})  [unwired: 1 in]
            n2022 = Bundle "Bundle"(w2313, w2341) -> (w2379:cluster{dbl[], dbl[]})  [unwired: 1 in]
            n2023 = Bundle "Bundle"(w2309, w2393) -> (w2401:cluster{dbl[], dbl[]})  [unwired: 1 in]
            n2024 = Bundle "Bundle"(w2311, w2394) -> (w2402:cluster{dbl[], dbl[]})  [unwired: 1 in]
            n2025 = Bundle "Bundle"(w2313, w2395) -> (w2403:cluster{dbl[], dbl[]})  [unwired: 1 in]
            n2026 = Bundle "Bundle"(w2313, w2434) -> (w2447:cluster{dbl[], dbl[]})  [unwired: 1 in]
            n2027 = Bundle "Bundle"(w2311, w2425) -> (w2449:cluster{dbl[], dbl[]})  [unwired: 1 in]
            n2028 = Bundle "Bundle"(w2309, w2416) -> (w2448:cluster{dbl[], dbl[]})  [unwired: 1 in]
            n2029 = Bundle "Bundle"(w2315, w2346) -> (w2333:cluster{dbl[], dbl[]})  [unwired: 1 in]
            n2030 = Bundle "Bundle"(w2313, w2345) -> (w2456:cluster{dbl[], dbl[]})  [unwired: 1 in]
            n2031 = Bundle "Bundle"(w2311, w2344) -> (w2454:cluster{dbl[], dbl[]})  [unwired: 1 in]
            n2032 = Bundle "Bundle"(w2309, w2343) -> (w2455:cluster{dbl[], dbl[]})  [unwired: 1 in]
            n2033 = Bundle "Bundle"(w2315, w2400) -> (w2334:cluster{dbl[], dbl[]})  [unwired: 1 in]
            n2034 = Bundle "Bundle"(w2313, w2397) -> (w2465:cluster{dbl[], dbl[]})  [unwired: 1 in]
            n2035 = Bundle "Bundle"(w2311, w2399) -> (w2464:cluster{dbl[], dbl[]})  [unwired: 1 in]
            n2036 = Bundle "Bundle"(w2309, w2398) -> (w2463:cluster{dbl[], dbl[]})  [unwired: 1 in]
            n2037 = call-poly <vilib>:"Mean.vi"("X"=w2397) -> ("mean"=→"КОФ2":dbl)  [unwired: 1 out]
            n2038 = call-poly <vilib>:"Mean.vi"("X"=w2398) -> ("mean"=→"КОФ4":dbl)  [unwired: 1 out]
            n2039 = call-poly <vilib>:"Mean.vi"("X"=w2396) -> ("mean"=→"CP1":dbl)  [unwired: 1 out]
            n2040 = call-poly <vilib>:"Mean.vi"("X"=w2395) -> ("mean"=→"CP2":dbl)  [unwired: 1 out]
            n2041 = call-poly <vilib>:"Mean.vi"("X"=w2393) -> ("mean"=→"CP4":dbl)  [unwired: 1 out]
            n2042 = call-poly <vilib>:"Mean.vi"("X"=w2337) -> ("mean"=→"КОФ2 3":dbl)  [unwired: 1 out]
            n2043 = call-poly <vilib>:"Mean.vi"("X"=w2335) -> ("mean"=→"КОФ2 5":dbl)  [unwired: 1 out]
            n2044 = Bundle "Bundle"(w2315, w2342) -> (w2306:cluster{dbl[], dbl[]})  [unwired: 1 in]
            n2045 = Bundle "Bundle"(w2315, w2396) -> (w2329:cluster{dbl[], dbl[]})  [unwired: 1 in]
            n2046 = Build Array "Build Array"(w2320, w2319, w2318, w2317) -> (→"Frequency ( Hz )":cluster{dbl[], dbl[]}[])
            n2047 = Build Array "Build Array"(w2306, w2329) -> (w2332:cluster{dbl[], dbl[]}[])
            "XY Graph 17" <- w2332
            n2048 = Build Array "Build Array"(w2348, w2349, w2350, w2351) -> (→"Air Temp ( °C ) vs Humidity ( % RH )":cluster{dbl[], dbl[]}[])
            n2049 = Build Array "Build Array"(w2306, w2379, w2378, w2377) -> (→"Humidity ( %RH )":cluster{dbl[], dbl[]}[])
            n2050 = Build Array "Build Array"(w2329, w2403, w2402, w2401) -> (→"Sample Temperature ( °C )":cluster{dbl[], dbl[]}[])
            n2051 = Build Array "Build Array"(w2307, w2447, w2449, w2448) -> (→"XY Graph 13":cluster{dbl[], dbl[]}[])
            n2052 = Build Array "Build Array"(w2333, w2456, w2454, w2455) -> (→"Air Temperature  ( °C )":cluster{dbl[], dbl[]}[])
            n2053 = Build Array "Build Array"(w2334, w2465, w2464, w2463) -> (→"Coefficient Of Friction":cluster{dbl[], dbl[]}[])
            n2054 = Bundle "Bundle"(w2309, w2335) -> (w2357:cluster{dbl[], dbl[]})  [unwired: 1 in]
            n2055 = Bundle "Bundle"(w2311, w2336) -> (w2358:cluster{dbl[], dbl[]})  [unwired: 1 in]
            n2056 = Bundle "Bundle"(w2313, w2337) -> (w2359:cluster{dbl[], dbl[]})  [unwired: 1 in]
            n2057 = Bundle "Bundle"(w2315, w2338) -> (w2360:cluster{dbl[], dbl[]})  [unwired: 1 in]
            n2058 = Build Array "Build Array"(w2360, w2359, w2358, w2357) -> (→"Stroke ( mm )":cluster{dbl[], dbl[]}[])
            n2059 = local write "XY Graph 16"(w2332) -> ()
          }
          frame #2 {
          }
          frame #3 {
            n2060 = local write "Numeric 8"(0 ("Numeric 8")) -> ()
            n2061 = local write "Numeric 11"(0 ("Numeric 11")) -> ()
            n2062 = local write "Numeric 12"(0 ("Numeric 12")) -> ()
            n2063 = local write "Numeric 13"(0 ("Numeric 13")) -> ()
            n2064 = property on="OPEN" class="Bool (strict)"("Visible"=TRUE) -> ()  [unwired: 2 in, 2 out]
            n2065 = local read "String Control 8"() -> (w2629:string)
            n2066 = local read "String Control 6"() -> (w2630:string)
            n2067 = local read "String Control 4"() -> (w2631:string)
            n2068 = local read "String Control 2"() -> (w2632:string)
            n2069 = Match Pattern(string=w2629, regular expression="Samples / cycle :- ") -> (after substring=w2634:string)  [unwired: 1 in, 3 out]
            n2070 = Match Pattern(string=w2630, regular expression="Samples / cycle :- ") -> (after substring=w2638:string)  [unwired: 1 in, 3 out]
            n2071 = Match Pattern(string=w2631, regular expression="Samples / cycle :- ") -> (after substring=w2642:string)  [unwired: 1 in, 3 out]
            n2072 = Match Pattern(string=w2632, regular expression="Samples / cycle :- ") -> (after substring=w2646:string)  [unwired: 1 in, 3 out]
            n2073 = Match Pattern(string=w2629, regular expression="Frequency :- ") -> (after substring=w2650:string)  [unwired: 1 in, 3 out]
            n2074 = Match Pattern(string=w2630, regular expression="Frequency :- ") -> (after substring=w2655:string)  [unwired: 1 in, 3 out]
            n2075 = Match Pattern(string=w2631, regular expression="Frequency :- ") -> (after substring=w2660:string)  [unwired: 1 in, 3 out]
            n2076 = Match Pattern(string=w2632, regular expression="Frequency :- ") -> (after substring=w2665:string)  [unwired: 1 in, 3 out]
            n2077 = String Subset(string=w2634, length (rest)=6 ("length (rest)")) -> (substring=w2636:string)  [unwired: 1 in]
            n2078 = String Subset(string=w2638, length (rest)=6 ("length (rest)")) -> (substring=w2640:string)  [unwired: 1 in]
            n2079 = String Subset(string=w2642, length (rest)=6 ("length (rest)")) -> (substring=w2644:string)  [unwired: 1 in]
            n2080 = String Subset(string=w2646, length (rest)=6 ("length (rest)")) -> (substring=w2648:string)  [unwired: 1 in]
            n2081 = String Subset(string=w2650, length (rest)=9 ("length (rest)")) -> (substring=w2652:string)  [unwired: 1 in]
            n2082 = String Subset(string=w2655, length (rest)=9 ("length (rest)")) -> (substring=w2657:string)  [unwired: 1 in]
            n2083 = String Subset(string=w2660, length (rest)=9 ("length (rest)")) -> (substring=w2662:string)  [unwired: 1 in]
            n2084 = String Subset(string=w2665, length (rest)=9 ("length (rest)")) -> (substring=w2667:string)  [unwired: 1 in]
            n2085 = Fract/Exp String To Number(string=w2636) -> (number=w2625:dbl)  [unwired: 3 in, 1 out]
            n2086 = Fract/Exp String To Number(string=w2640) -> (number=w2626:dbl)  [unwired: 3 in, 1 out]
            n2087 = Fract/Exp String To Number(string=w2644) -> (number=w2627:dbl)  [unwired: 3 in, 1 out]
            n2088 = Fract/Exp String To Number(string=w2648) -> (number=w2628:dbl)  [unwired: 3 in, 1 out]
            n2089 = Fract/Exp String To Number(string=w2652) -> (number=w2653:dbl)  [unwired: 3 in, 1 out]
            n2090 = Fract/Exp String To Number(string=w2657) -> (number=w2658:dbl)  [unwired: 3 in, 1 out]
            n2091 = Fract/Exp String To Number(string=w2662) -> (number=w2663:dbl)  [unwired: 3 in, 1 out]
            n2092 = Fract/Exp String To Number(string=w2667) -> (number=w2668:dbl)  [unwired: 3 in, 1 out]
            n2093 = local write "sample4"(w2625) -> ()
            n2094 = local write "sample3"(w2626) -> ()
            n2095 = local write "sample2"(w2627) -> ()
            n2096 = local write "sample1"(w2628) -> ()
            n2097 = local write "freq 4"(w2653) -> ()
            n2098 = local write "freq3"(w2658) -> ()
            n2099 = local write "freq2"(w2663) -> ()
            n2100 = local write "freq1"(w2668) -> ()
          }
        }
      }
    }
    n2101 = case shown="True" w2226 {
      selector: w2226 -> [_ w2245]
      frame False {
      }
      frame True {
        n2102 = Not(x=w2245) -> (.not. x?=w2241:bool)
        n2103 = local write "service 3"(w2241) -> ()
        n2104 = local write "OPEN 6"(w2241) -> ()
        n2105 = call <vilib>:"System Exec.vi"("wait until completion? (T)"=TRUE, "command line"="C:\\LAB-IQ\\Scar View.exe") -> ("error out"=→"error out 5":errorcluster)  [unwired: 6 in, 3 out]
      }
    }
    n2106 = flat-sequence {
      frame #0 {
        n2107 = local read "x = y?"() -> (w2716:bool)
        n2108 = And(x="EDIT", y=w2716) -> (x .and. y?=w2714:bool)
        n2109 = stacked-sequence {
          frame #0 {
            n2110 = local read "EDIT"() -> (w2718:bool)
            n2111 = case shown="False" w2718 {
              tunnel: [u8 2 ("Disabled") u8 0 ("Disabled")] -> _
              frame False {
                w2720 = FALSE
                n2112 = local write "Password"("") -> ()
                n2113 = local write "x = y?"(w2720) -> ()
                n2114 = property on="Password" class="Str"("Visible"=w2720) -> ()  [unwired: 2 in, 2 out]
              }
              frame True {
                n2115 = property on="Password" class="Str"("Visible"=TRUE) -> ()  [unwired: 2 in, 2 out]
              }
            }
            "dipl pwd" <- "@143$\n" ("dipl pwd")
          }
          frame #1 {
          }
          frame #2 {
          }
          frame #3 {
          }
          frame #4 {
            n2116 = String To Byte Array(string="Password") -> (unsigned byte array=w2731:u8[])
            n2117 = Search 1D Array(1D array=w2731, element=u8 10) -> (index of element=w2729:i32)  [unwired: 1 in]
            n2118 = Index Array(array=w2731, index=w2729) -> (element=w2730:u8)
            n2119 = Equal?(x=w2730, y=10) -> (x = y?=w2726:bool)
            n2120 = case shown="True" w2726 {
              frame False {
              }
              frame True {
                # "password"
                # "password"
                n2121 = local read "Password"() -> (w2743:string)
                n2122 = String To Byte Array(string="@143$\n") -> (unsigned byte array=w2733:u8[])
                n2123 = String To Byte Array(string=w2743) -> (unsigned byte array=w2746:u8[])
                n2124 = Array Size(array=w2733) -> (size(s)=w2738:i32)
                n2125 = Array Size(array=w2746) -> (size(s)=w2742:i32)
                n2126 = for {
                  N: w2742 -> [_]
                  tunnel: w2746 -> [w2759]
                  tunnel: [w2757] -> w2747 mode=indexing
                  tunnel: w2742 -> [w2754]
                  i -> [w2755]
                  n2127 = Decrement(x=w2754) -> (x-1=w2753:i32)
                  n2128 = Equal?(x=w2755, y=w2753) -> (x = y?=w2752:bool)
                  n2129 = Index Array(array=w2759, index=w2755) -> (element=w2758:u8)
                  n2130 = Number To Decimal String(number=w2758) -> (decimal integer string=w2756:string)  [unwired: 1 in]
                  n2131 = Select(t="", s=w2752, f="\r") -> (s? t:f=w2749:string)
                  n2132 = Concatenate Strings(w2756, w2749) -> (w2757:string)
                }
                n2133 = for {
                  N: w2738 -> [_]
                  tunnel: w2733 -> [w2770]
                  tunnel: [w2768] -> w2736 mode=indexing
                  tunnel: w2738 -> [w2765]
                  i -> [w2766]
                  n2134 = Decrement(x=w2765) -> (x-1=w2764:i32)
                  n2135 = Equal?(x=w2766, y=w2764) -> (x = y?=w2763:bool)
                  n2136 = Index Array(array=w2770, index=w2766) -> (element=w2769:u8)
                  n2137 = Number To Decimal String(number=w2769) -> (decimal integer string=w2767:string)  [unwired: 1 in]
                  n2138 = Select(t="", s=w2763, f="\r") -> (s? t:f=w2760:string)
                  n2139 = Concatenate Strings(w2767, w2760) -> (w2768:string)
                }
                n2140 = local read "file path"() -> (w2732:path)
                n2141 = call <vilib>:"Read Characters From File.vi"("file path (dialog if empty)"=w2732) -> ("character string"=w2745:string)  [unwired: 5 in, 3 out]
                "string" <- w2745
                n2142 = flat-sequence {
                  tunnel: [w2748] -> _
                  frame #0 {
                    w2748 = ""
                    n2143 = local write "Password"(w2748) -> ()
                  }
                }
                n2144 = Concatenate Strings(w2736) -> (w2737:string)
                n2145 = Concatenate Strings(w2745) -> (w2744:string)
                n2146 = Concatenate Strings(w2747) -> (w2740:string)
                n2147 = Equal?(x=w2740, y=w2737) -> (x = y?=w2741:bool)
                n2148 = Equal?(x=w2740, y=w2744) -> (x = y?=w2735:bool)
                n2149 = Or(x=w2735, y=w2741) -> (x .or. y?=→"x = y?":bool)
              }
            }
          }
        }
        n2150 = case shown="True" w2714 {
          tunnel: [u8 2 ("Disabled") u8 0 ("Disabled")] -> w2713
          tunnel: [w2920 TRUE ("Visible")] -> w2712
          frame False {
            w2920 = FALSE ("Visible")
            n2151 = local write "EDIT 2"(w2920) -> ()
          }
          frame True {
          }
        }
        n2152 = property on="EDIT 2" class="Bool (strict)"("Visible"=w2712) -> ()  [unwired: 2 in, 2 out]
        n2153 = property on="File Path" class="Path"("Disabled"=w2713) -> ()  [unwired: 2 in, 2 out]
        n2154 = property on="visa due" class="CmbBox"("Disabled"=w2713) -> ()  [unwired: 2 in, 2 out]
        n2155 = property on="SAVE" class="Bool (strict)"("Visible"=w2712) -> ()  [unwired: 2 in, 2 out]
        n2156 = case shown="True" "SAVE" {
          frame False {
          }
          frame True {
            n2157 = stacked-sequence {
              seq-local: [w2775 _ _] -> [_ w2916 _]
              frame #0 {
                w2771 = 0.0 ("number")
                w2772 = 0.0 ("number")
                (unwired) i16 5 ("precision (6)")
                # "[CH1]    - FF\n[CH2]   - TEMPERATURE\n[CH3]    - Humidity\n[CH4]    - AIR TEMP\n[CH5]\\- Visa Uno\n[CH6] \\- Visa Due\n[CH7]  \\- file path\n[CH8]   - Displacement Gain\n[CHA]   - Stroke Gain\n[CHB]   - Stroke PID Gain\n[CHC]   -Language Selection\n[CHD]   -Power +\n[CHE]   -Power_\n[CHF]   -Heater\n[CHG]   -Humidity Wet\n[CHH]   -Humidity Dry\n[CHI]   -Integral Time"
                n2158 = local read "Language Selection"() -> (w2818:enum16{"English", "Russian"})
                n2159 = Path To String(path="File Path") -> (string=w2834:string)
                n2160 = Number To Fractional String(number=w2772, width (-)=i16 10 ("precision (6)"), precision (6)=i16 5) -> (F-format string=w2792:string)  [unwired: 1 in]
                n2161 = Number To Fractional String(number=w2772, width (-)=i16 10 ("precision (6)"), precision (6)=i16 5) -> (F-format string=w2797:string)  [unwired: 1 in]
                n2162 = Number To Fractional String(number=w2772, width (-)=i16 10 ("precision (6)"), precision (6)=i16 5) -> (F-format string=w2800:string)  [unwired: 1 in]
                n2163 = Number To Fractional String(number=w2772, width (-)=i16 10 ("precision (6)"), precision (6)=i16 5) -> (F-format string=w2805:string)  [unwired: 1 in]
                n2164 = Number To Fractional String(number=w2772, width (-)=i16 10 ("precision (6)"), precision (6)=i16 5) -> (F-format string=w2808:string)  [unwired: 1 in]
                n2165 = Number To Fractional String(number=w2818, width (-)=i16 10 ("precision (6)"), precision (6)=i16 5) -> (F-format string=w2814:string)  [unwired: 1 in]
                n2166 = Number To Fractional String(number=w2771, width (-)=i16 10 ("precision (6)"), precision (6)=i16 5) -> (F-format string=w2825:string)  [unwired: 1 in]
                n2167 = local read "Com Port 2"() -> (w2773:refnum<visa-resource-name>)
                n2168 = local read "Com Port 1"() -> (w2774:refnum<visa-resource-name>)
                n2169 = Concatenate Strings(w2834, "\\" ("string")) -> (w2833:string)
                n2170 = Number To Fractional String(number=w2771, width (-)=i16 10 ("precision (6)"), precision (6)=i16 5) -> (F-format string=w2826:string)  [unwired: 1 in]
                n2171 = Number To Fractional String(number=w2771, width (-)=i16 10 ("precision (6)"), precision (6)=i16 5) -> (F-format string=w2853:string)  [unwired: 1 in]
                n2172 = Number To Fractional String(number=w2771, width (-)=i16 10 ("precision (6)"), precision (6)=i16 5) -> (F-format string=w2859:string)  [unwired: 1 in]